vi "HFRR ADV v044.vi"() -> ()   [LabVIEW 2025] (continued)
                  n3206 = call-dynamic "Set Report Tab Width.vi"("report in"=w4016, "error in (no error)"=w4014) -> ("report out"=w4015:refnum<class "NI_report.lvclass">, "error out"=w4013:errorcluster)  [unwired: 12 in]
                }
                n3207 = local read "TITTLE"() -> (w3961:string)
                n3208 = call-dynamic "Set Report Header Text.vi"("report in"=w3944, "center header text"=w3961, "error in (no error)"=w3943) -> ("report out"=w3982:refnum<class "NI_report.lvclass">, "error out"=w3981:errorcluster)  [unwired: 11 in]
                n3209 = for {
                  N: 1 -> [_]
                  tunnel: [w4020] -> w3968
                  tunnel: [w4019] -> w3967
                  tunnel: w3982 -> [w4018]
                  tunnel: w3981 -> [w4017]
                  n3210 = call-dynamic "New Report Line.vi"("report in"=w4018, "error in (no error)"=w4017) -> ("report out"=w4020:refnum<class "NI_report.lvclass">, "error out"=w4019:errorcluster)  [unwired: 12 in]
                }
                n3211 = for {
                  N: 2 -> [_]
                  tunnel: [w4012] -> w3974
                  tunnel: [w4011] -> w3973
                  tunnel: w3968 -> [w4010]
                  tunnel: w3967 -> [w4009]
                  n3212 = call-dynamic "New Report Line.vi"("report in"=w4010, "error in (no error)"=w4009) -> ("report out"=w4012:refnum<class "NI_report.lvclass">, "error out"=w4011:errorcluster)  [unwired: 12 in]
                }
                n3213 = for {
                  N: 25 -> [_]
                  tunnel: w3974 -> [w4008]
                  tunnel: w3973 -> [w4006]
                  tunnel: [w4007] -> w3977
                  tunnel: [w4005] -> w3976
                  n3214 = call-dynamic "Set Report Tab Width.vi"("report in"=w4008, "error in (no error)"=w4006) -> ("report out"=w4007:refnum<class "NI_report.lvclass">, "error out"=w4005:errorcluster)  [unwired: 12 in]
                }
                n3215 = control-ref of="Tab Control 9"() -> (w3972:refnum<vi>)
                n3216 = call-dynamic "Append Control Image to Report.vi"("report in"=w3977, "alignment (default)"=HTML_Report_Image_Alignment."ABSMIDDLE", "ctrl reference"=w3972, "error in (no error)"=w3976) -> ("report out"=w3971:refnum<class "NI_report.lvclass">, "error out"=w3970:errorcluster)  [unwired: 8 in, 2 out]
                n3217 = for {
                  N: 3 -> [_]
                  tunnel: [w4004] -> w3955
                  tunnel: [w4003] -> w3954
                  tunnel: w3971 -> [w4002]
                  tunnel: w3970 -> [w4001]
                  n3218 = call-dynamic "New Report Line.vi"("report in"=w4002, "error in (no error)"=w4001) -> ("report out"=w4004:refnum<class "NI_report.lvclass">, "error out"=w4003:errorcluster)  [unwired: 12 in]
                }
                n3219 = for {
                  N: 100 -> [_]
                  tunnel: w3955 -> [w4000]
                  tunnel: w3954 -> [w3998]
                  tunnel: [w3999] -> w3951
                  tunnel: [w3997] -> w3949
                  n3220 = call-dynamic "Set Report Tab Width.vi"("report in"=w4000, "error in (no error)"=w3998) -> ("report out"=w3999:refnum<class "NI_report.lvclass">, "error out"=w3997:errorcluster)  [unwired: 12 in]
                }
                n3221 = String To Path(string="C:\\LAB-IQ\\im\\Temp_resized.jpg") -> (path=w3941:path)
                n3222 = call-poly <vilib>:"Append Image to Report.vi"("report in"=w3951, "path or URL of image"=w3941, "error in (no error)"=w3949) -> ("report out"=w3950:refnum<class "NI_report.lvclass">, "error out"=w3948:errorcluster)  [unwired: 9 in, 2 out]
                n3223 = call-poly <vilib>:"Open HTML Report in Browser.vi"("report in"=w3950, "error in (no error)"=w3948) -> ("report out"=w3985:refnum<class "NI_report.lvclass">, "error out"=w3984:errorcluster)  [unwired: 11 in, 1 out]
                n3224 = call-dynamic "Dispose Report.vi"("report in"=w3985, "error in (no error)"=w3984) -> ()  [unwired: 13 in, 1 out]
              }
              frame #2 {
              }
              frame #3 {
                n3225 = disable-structure shown="Disabled" {
                  frame Disabled {
                    n3226 = local read "String 10"() -> (w4025:string)
                    n3227 = Concatenate Strings("C:\\LAB-IQ-NXT\\Data\\" ("string"), w4025, ".jpg" ("string")) -> (w4023:string)
                    n3228 = String To Path(string=w4023) -> (path=w4022:path)
                    n3229 = Delete(path (use dialog)=w4022) -> ()  [unwired: 4 in, 3 out]
                  }
                  frame Enabled {
                  }
                }
                n3230 = local write "Print 2"(FALSE ("Print")) -> ()
              }
            }
          }
        }
      }
    }
    n3231 = Wait (ms)(milliseconds to wait=u32 50) -> ()  [unwired: 1 out]
    n3232 = Wait (ms)(milliseconds to wait=u32 50) -> ()  [unwired: 1 out]
    n3233 = local read "Quit"() -> (w2367:bool)
  }
  n3234 = VISA Close(VISA resource name=w46, error in (no error)=w45) -> ()  [unwired: 1 out]
  n3235 = while {
    stop <- w4176 stop-if-true
    n3236 = local read "Auto Start Test"() -> (w4174:bool)
    n3237 = local read "RUN"() -> (w4173:bool)
    n3238 = Wait (ms)(milliseconds to wait=u32 1000) -> ()  [unwired: 1 out]
    n3239 = Or(x=w4173, y=w4174) -> (x .or. y?=w4172:bool)
    n3240 = case shown="True" w4172 {
      frame False {
      }
      frame True {
        n3241 = local read "LVDT STROKE Actual"() -> (w4177:dbl)
        n3242 = In Range and Coerce(upper limit=1.2, x=w4177, lower limit=0.6) -> (In Range?=w4180:bool)  [unwired: 1 out]
        n3243 = call-poly <vilib>:"Random Number (Range).vi"("lower bound (0)"=0.998 ("upper bound (100)"), "upper bound (100)"=1.003) -> ("number"=w4178:dbl)  [unwired: 9 in]
        n3244 = case shown="True" w4180 {
          tunnel: [w4185 w4186] -> w4179
          tunnel: w4178 -> [_ w4186]
          tunnel: w4177 -> [w4185 _]
          frame False {
          }
          frame True {
          }
        }
        "LVDT STROKE DISPLAY" <- w4179
      }
    }
    n3245 = local read "Quit"() -> (w4176:bool)
  }
  n3246 = while {
    tunnel: [w4203] -> w54
    shift-right: [w4196] -> _
    shift-left: 0.0 -> [w4199]
    shift-right: [w4195] -> _
    shift-left: 0.0 -> [w4198]
    shift-right: [w4194] -> _
    shift-left: 100.0 ("vc_cmd") -> [w4197]
    stop <- w4203 stop-if-true
    # "PID LOGIC"
    n3247 = local read "run test Calibration"() -> (w4191:bool)
    n3248 = local read "RUN"() -> (w4201:bool)
    n3249 = local read "Auto Start Temp"() -> (w4192:bool)
    n3250 = local read "Auto Start Test"() -> (w4200:bool)
    n3251 = local read "START TEMP"() -> (w4190:bool)
    n3252 = And(x=w4192, y=w4200) -> (x .and. y?=w4193:bool)
    n3253 = Or(x=w4201, y=w4193) -> (x .or. y?=w4202:bool)
    n3254 = And(x=w4202, y=w4190) -> (x .and. y?=w4189:bool)
    n3255 = And(x=w4191, y=w4190) -> (x .and. y?=w4188:bool)
    n3256 = Or(x=w4188, y=w4189) -> (x .or. y?=w4187:bool)
    n3257 = Wait (ms)(milliseconds to wait="milliseconds to wait") -> ()  [unwired: 1 out]
    n3258 = case shown="True" w4187 {
      tunnel: [400.0 ("out_vc_cmd") w4222] -> w4194
      tunnel: [w4206 w4224] -> w4195
      tunnel: [w4206 w4223] -> w4196
      tunnel: w4199 -> [_ w4213]
      tunnel: w4198 -> [_ w4212]
      tunnel: w4197 -> [_ w4211]
      tunnel: w4191 -> [_ w4207]
      frame False {
        w4206 = 0.0 ("error_out")
      }
      frame True {
        n3259 = case shown="True" w4207 {
          tunnel: [w4231 1.0] -> w4209
          frame False {
            n3260 = local read "Set Strk"() -> (w4230:dbl)
            n3261 = Add(x=w4230, y="Add up Stroke") -> (x+y=w4231:dbl)
          }
          frame True {
          }
        }
        n3262 = local read "LVDT STROKE"() -> (w4208:dbl)
        n3263 = formula code="// Zero-Hardcode Explicit Positional-Form PID Engine\n// Inputs: target_stroke, measured_stroke, dt, prev_error, integral_accumulator_in, prev_vc_cmd\n//         kp, ki, kd, max_step_change, max_amplitude, min_amplitude, startup_cmd\n// Outputs: vc_cmd, error_out, out_error, integral_accumulator_out, out_vc_cmd\n\n// 1. Calculate Tracking Error\nfloat current_error = target_stroke - measured_stroke;\nerror_out = current_error;\n\n// 2. Compute Proportional Term\nfloat p_term = kp * current_error;\n\n// 3. Compute Derivative Term\nfloat d_term = 0.0;\nif (dt > 0.0) {\n    d_term = kd * ((current_error - prev_error) / dt);\n}\n\n// 4. Update and Accumulate Integral Term\nfloat current_integral = integral_accumulator_in + (current_error * dt);\nfloat i_term = ki * current_integral;\n\n// 5. Calculate Ideal Target Command (Anchored by startup baseline)\nfloat ideal_command = startup_cmd + p_term + i_term + d_term;\n\n// 6. Apply Loop Rate Limiting FIRST \n// (Forces the command to climb gradually from prev_vc_cmd instead of jumping straight to max)\nfloat raw_adjustment = ideal_command - prev_vc_cmd;\n\nif (raw_adjustment > max_step_change) {\n    raw_adjustment = max_step_change;\n} else if (raw_adjustment < -max_step_change) {\n    raw_adjustment = -max_step_change;\n}\n\nfloat next_vc_cmd = prev_vc_cmd + raw_adjustment;\n\n// 7. Anti-Windup Protection & Final Output Safety Safeguard Clamping\n// (Back-calculating based on what we are ACTUALLY outputting)\nif (next_vc_cmd > max_amplitude) {\n    float excess = next_vc_cmd - max_amplitude;\n    if (ki > 0.0) {\n        current_integral -= excess / ki;\n    }\n    next_vc_cmd = max_amplitude;\n} else if (next_vc_cmd < min_amplitude) {\n    float excess = next_vc_cmd - min_amplitude;\n    if (ki > 0.0) {\n        current_integral -= excess / ki;\n    }\n    next_vc_cmd = min_amplitude;\n}\n\n// 8. Map to Shift Registers for memory persistence\nvc_cmd = next_vc_cmd;\nout_error = current_error;                   \nintegral_accumulator_out = current_integral;  \nout_vc_cmd = next_vc_cmd;"("target_stroke"=w4209, "measured_stroke"=w4208, "dt"="dt", "integral_accumulator_in"=w4212, "prev_error"=w4213, "prev_vc_cmd"=w4211, "kp"="kp", "ki"="ki", "kd"="kd", "max_step_change"="max_step_change", "max_amplitude"="max_amplitude", "min_amplitude"="min_amplitude", "startup_cmd"="startup_cmd") -> ("vc_cmd"=w4228:dbl, "out_error"=w4223:dbl, "integral_accumulator_out"=w4224:dbl, "out_vc_cmd"=w4222:dbl)  [unwired: 1 out]
        "output Vpp" <- w4228
        n3264 = Number To Fractional String(number=w4228, precision (6)=i16 1) -> (F-format string=w4226:string)  [unwired: 2 in]
        n3265 = Concatenate Strings("DAC;" ("string"), w4226) -> (w4210:string)
        n3266 = local write "Due Write"(w4210) -> ()
        "prev_error" <- w4213
        "integral_accumulator_in" <- w4212
        "prev_vc_cmd" <- w4211
      }
    }
    n3267 = local read "Quit"() -> (w4203:bool)
  }
  n3268 = Or(x=w50, y=w49) -> (x .or. y?=w51:bool)
  n3269 = Or(x=w47, y=w51) -> (x .or. y?=w56:bool)
  n3270 = control-ref of="new picture"() -> ()  [unwired: 1 out]
  n3271 = Or(x=w59, y=w56) -> (x .or. y?=w53:bool)
  n3272 = Or(x=w53, y=w54) -> (x .or. y?=w48:bool)
  n3273 = while {
    tunnel: [w4233] -> w58
    i -> [w4240]
    stop <- w4233 stop-if-true
    n3274 = local read "Quit"() -> (w4233:bool)
    n3275 = Equal To 0?(x=w4240) -> (x = 0?=w4238:bool)
    n3276 = call "Elapsed Time3"("Time Target (s)"=45.0, "Auto Reset"=TRUE) -> ("Time has Elapsed"=w4237:bool)  [unwired: 10 in, 7 out]
    n3277 = Wait (ms)(milliseconds to wait=u32 50) -> ()  [unwired: 1 out]
    n3278 = Or(x=w4237, y=w4238) -> (x .or. y?=w4239:bool)
    n3279 = case shown="True" w4239 {
      frame False {
      }
      frame True {
        n3280 = call <vilib>:"System Exec.vi"("run minimized? (F)"=TRUE, "error in (no error)"="error in (no error)", "command line"="powercfg.exe -change -monitor-timeout-ac 0") -> ("error out"=w4251:errorcluster)  [unwired: 5 in, 3 out]
        n3281 = call <vilib>:"System Exec.vi"("run minimized? (F)"=TRUE, "error in (no error)"=w4251, "command line"="powercfg.exe -change -disk-timeout-ac 0") -> ("error out"=w4250:errorcluster)  [unwired: 5 in, 3 out]
        n3282 = call <vilib>:"System Exec.vi"("run minimized? (F)"=TRUE, "error in (no error)"=w4250, "command line"="powercfg.exe -change -standby-timeout-ac 0") -> ("error out"=w4249:errorcluster)  [unwired: 5 in, 3 out]
        n3283 = call <vilib>:"System Exec.vi"("run minimized? (F)"=TRUE, "error in (no error)"=w4249, "command line"="powercfg.exe -change -hibernate-timeout-ac 0") -> ("error out"=w4248:errorcluster)  [unwired: 5 in, 3 out]
        n3284 = call <vilib>:"Simple Error Handler.vi"("error in (no error)"=w4248) -> ("error out"=w4254:errorcluster)  [unwired: 4 in, 4 out]
        n3285 = call <vilib>:"Clear Errors.vi"("error in (no error)"=w4254) -> ("error out"=→"error out":errorcluster)  [unwired: 5 in, 1 out]
      }
    }
  }
  n3286 = Compound Arithmetic op=OR(w61, w48, w58) -> (w60:bool)
  n3287 = flat-sequence {
    tunnel: w60 -> [_]
    tunnel: [w4256] -> w30
    tunnel: w30 -> [_]
    frame #0 {
      n3288 = call "CLOSE CONNECTION.vi"() -> ("error out"=w4256:errorcluster)  [unwired: 11 in]
    }
    frame #1 {
      n3289 = Quit LabVIEW(quit? (T)=TRUE) -> ()
      n3290 = local write "Quit"(FALSE ("EXIT")) -> ()
    }
  }
  n3291 = property on="Heater Button" class="Bool (strict)"("Visible"=TRUE) -> ()  [unwired: 2 in, 2 out]
  n3292 = while {
    tunnel: [w4263] -> _
    i -> [w4263]
    stop <- w4259 stop-if-true
    # "Langauage selection"
    n3293 = Equal?(x="Lan flag", y=22.0) -> ()  [unwired: 1 out]
    n3294 = disable-structure shown="Disabled" {
      frame Disabled {
        n3295 = stacked-sequence {
          frame #0 {
            n3296 = case shown="\"Russian\"" "Language Selection" {
              tunnel: [0 1] -> w4265
              frame "English", Default {
              }
              frame "Russian" {
              }
            }
            n3297 = for {
              N: 130 -> [_]
              tunnel: "Table" -> [w4274]
              tunnel: w4265 -> [w4273]
              i -> [w4272]
              n3298 = Index Array(array=w4274, index (row)=w4272, index (col)=w4273) -> (element=w4271:string)
              n3299 = case shown="1" w4272 {
                tunnel: w4271 -> [w4275 w4276 _ w4277 w4278 w4279 w4280 w4281 w4282 w4283 w4284 w4285 w4286 w4287 w4288 w4289 w4290 w4291 w4292 w4293 w4294 w4295 w4296 w4297 w4298 w4299 w4300 w4301 w4302 _ _ w4303 w4304 w4305 w4306 w4307 w4308 w4317 w4324 w4331 w4338 w4342 w4345 w4348 w4350 w4352 w4353 w4354 w4355 w4356 w4357 w4358 w4359 w4360 w4361 w4362 w4363 w4364 w4365 w4366 w4367 w4368 w4369 w4370 w4371 w4372 w4373 w4374 w4375 w4376 w4377 w4378 w4379 w4380 w4381 w4382 w4383 w4384 w4385 w4386 w4387 w4388 w4389 w4390 w4391 w4392 w4393 w4394 w4395 w4396 w4397 w4398 w4399 w4400 w4401 w4402 w4403 w4404 w4405 w4406 w4407 w4408 w4409 w4410 w4411 _ w4412 w4413 w4414 w4415 w4416 w4417 w4418 w4419 w4420 w4421 w4422 w4423 w4424 _ w4425 w4426 w4427 w4428 w4429 w4430 _]
                frame 0 {
                  n3300 = local write "S"(w4275) -> ()
                }
                frame 1 {
                  n3301 = local write "S 2"(w4276) -> ()
                }
                frame 2 {
                }
                frame 3 {
                  n3302 = local write "S 4"(w4277) -> ()
                }
                frame 4 {
                  n3303 = property on="FILE" class="Str"("Caption.Text"=w4278) -> ()  [unwired: 2 in, 2 out]
                }
                frame 5 {
                  n3304 = property on="Fuel Discription :" class="Str"("Caption.Text"=w4279) -> ()  [unwired: 2 in, 2 out]
                }
                frame 6 {
                  n3305 = property on="Remarks :" class="Str"("Caption.Text"=w4280) -> ()  [unwired: 2 in, 2 out]
                }
                frame 7 {
                  n3306 = property on="Save & Continue" class="Bool (strict)"("Boolean Text.Text"=w4281) -> ()  [unwired: 2 in, 2 out]
                }
                frame 8 {
                }
                frame 9 {
                  n3307 = property on="Set Hz" class="DigNum (strict)"("Caption.Text"=w4283) -> ()  [unwired: 2 in, 2 out]
                }
                frame 10 {
                }
                frame 11 {
                  n3308 = property on="NORMAL LOAD" class="DigNum (strict)"("Caption.Text"=w4285) -> ()  [unwired: 2 in, 2 out]
                }
                frame 12 {
                }
                frame 13 {
                  n3309 = property on="Set Temp" class="DigNum (strict)"("Caption.Text"=w4287) -> ()  [unwired: 2 in, 2 out]
                }
                frame 14 {
                  n3310 = local write "S 15"(w4288) -> ()
                }
                frame 15 {
                  n3311 = property on="Set Rh" class="DigNum (strict)"("Caption.Text"=w4289) -> ()  [unwired: 2 in, 2 out]
                }
                frame 16 {
                }
                frame 17 {
                  n3312 = local write "S 18"(w4291) -> ()
                }
                frame 18 {
                  "String 17" <- w4292
                }
                frame 19 {
                  n3313 = property on="test time" class="DigNum (strict)"("Caption.Text"=w4293) -> ()  [unwired: 2 in, 2 out]
                }
                frame 20 {
                  "String 18" <- w4294
                  "String 22" <- w4294
                }
                frame 21 {
                  n3314 = property on="Elapsed time" class="DigNum (strict)"("Caption.Text"=w4295) -> ()  [unwired: 2 in, 2 out]
                }
                frame 22 {
                  n3315 = property on="Samplingtime 2" class="DigNum (strict)"("Caption.Text"=w4296) -> ()  [unwired: 2 in, 2 out]
                }
                frame 23 {
                  "String 21" <- w4297
                }
                frame 24 {
                  n3316 = property on="Countdown" class="DigNum (strict)"("Caption.Text"=w4298) -> ()  [unwired: 2 in, 2 out]
                }
                frame 25 {
                  n3317 = property on="Countdown 2" class="DigNum (strict)"("Caption.Text"=w4299) -> ()  [unwired: 2 in, 2 out]
                }
                frame 26 {
                  n3318 = property on="Engage" class="Bool (strict)"("Boolean Text.Text"=w4300) -> ()  [unwired: 2 in, 2 out]
                }
                frame 27 {
                  n3319 = property on="Boolean  4" class="Bool (strict)"("Boolean Text.Text"=w4301) -> ()  [unwired: 2 in, 2 out]
                }
                frame 28 {
                  n3320 = property on="Test \nStatus" class="Bool (strict)"("Boolean Text.Text"=w4302) -> ()  [unwired: 2 in, 2 out]
                }
                frame 29 {
                }
                frame 30 {
                }
                frame 31 {
                }
                frame 32 {
                  n3321 = property on="RSTCOF" class="Bool"("Boolean Text.Text"=w4304) -> ()  [unwired: 2 in, 2 out]
                  n3322 = property on="RST FF" class="Bool"("Boolean Text.Text"=w4304) -> ()  [unwired: 2 in, 2 out]
                  n3323 = property on="RST TEMP" class="Bool"("Boolean Text.Text"=w4304) -> ()  [unwired: 2 in, 2 out]
                  n3324 = property on="RSTV1 3" class="Bool"("Boolean Text.Text"=w4304) -> ()  [unwired: 2 in, 2 out]
                  n3325 = property on="rstv2" class="Bool"("Boolean Text.Text"=w4304) -> ()  [unwired: 2 in, 2 out]
                  n3326 = property on="RSTV1 2" class="Bool"("Boolean Text.Text"=w4304) -> ()  [unwired: 2 in, 2 out]
                  n3327 = property on="RST CP" class="Bool"("Boolean Text.Text"=w4304) -> ()  [unwired: 2 in, 2 out]
                }
                frame 33 {
                  "S 61" <- w4305
                }
                frame 34 {
                  "String 23" <- w4306
                }
                frame 35 {
                  n3328 = property on="Rh Before" class="DigNum (strict)"("Caption.Text"=w4307) -> ()  [unwired: 2 in, 2 out]
                }
                frame 36 {
                  n3329 = Match Pattern(string=w4308, regular expression=",") -> (before substring=→"bs":string, after substring=→"as":string)  [unwired: 1 in, 2 out]
                  n3330 = property on="Rh After" class="DigNum (strict)"("Caption.Text"=w4308) -> ()  [unwired: 2 in, 2 out]
                }
                frame 37 {
                  n3331 = Match Pattern(string=w4317, regular expression=",") -> (before substring=w4316:string, after substring=w4315:string)  [unwired: 1 in, 2 out]
                  "bs" <- w4316
                  "as" <- w4315
                  n3332 = Concatenate Strings(w4316, w4315) -> (w4312:string)
                  n3333 = property on="Humidity before test 2" class="DigNum (strict)"("Caption.Text"=w4312) -> ()  [unwired: 2 in, 2 out]
                  n3334 = Concatenate Strings(w4312, "=" ("string")) -> (w4313:string)
                  n3335 = local write "S 38"(w4313) -> ()
                }
                frame 38 {
                  n3336 = Match Pattern(string=w4324, regular expression=",") -> (before substring=w4323:string, after substring=w4322:string)  [unwired: 1 in, 2 out]
                  "bs" <- w4323
                  "as" <- w4322
                  n3337 = Concatenate Strings(w4323, w4322) -> (w4319:string)
                  n3338 = property on="Humidity after test 2" class="DigNum (strict)"("Caption.Text"=w4319) -> ()  [unwired: 2 in, 2 out]
                  n3339 = Concatenate Strings(w4319, "=" ("string")) -> (w4321:string)
                  n3340 = local write "S 39"(w4321) -> ()
                }
                frame 39 {
                  n3341 = Match Pattern(string=w4331, regular expression=",") -> (before substring=w4330:string, after substring=w4329:string)  [unwired: 1 in, 2 out]
                  "bs" <- w4330
                  "as" <- w4329
                  n3342 = Concatenate Strings(w4330, w4329) -> (w4326:string)
                  n3343 = property on="Temperature before test 2" class="DigNum (strict)"("Caption.Text"=w4326) -> ()  [unwired: 2 in, 2 out]
                  n3344 = Concatenate Strings(w4326, "=" ("string")) -> (→"String 34":string)
                }
                frame 40 {
                  n3345 = Match Pattern(string=w4338, regular expression=",") -> (before substring=w4337:string, after substring=w4336:string)  [unwired: 1 in, 2 out]
                  "bs" <- w4337
                  "as" <- w4336
                  n3346 = Concatenate Strings(w4337, w4336) -> (w4333:string)
                  n3347 = property on="Temperature after test 2" class="DigNum (strict)"("Caption.Text"=w4333) -> ()  [unwired: 2 in, 2 out]
                  n3348 = Concatenate Strings(w4333, "=" ("string")) -> (→"String 35":string)
                  n3349 = property on="Temperature after test" class="DigNum (strict)"("Caption.Text"=w4333) -> ()  [unwired: 2 in, 2 out]
                }
                frame 41 {
                  n3350 = property on="AVP 2" class="DigNum (strict)"("Caption.Text"=w4342) -> ()  [unwired: 2 in, 2 out]
                  n3351 = Concatenate Strings(w4342, "=" ("string")) -> (→"String 36":string)
                }
                frame 42 {
                  n3352 = property on="MWSD 2" class="DigNum (strict)"("Caption.Text"=w4345) -> ()  [unwired: 2 in, 2 out]
                  n3353 = Concatenate Strings(w4345, "=" ("string")) -> (→"String 37":string)
                }
                frame 43 {
                  n3354 = property on="HCF 2" class="DigNum (strict)"("Caption.Text"=w4348) -> ()  [unwired: 2 in, 2 out]
                  n3355 = Concatenate Strings(w4348, "=" ("string")) -> (→"String 38":string)
                }
                frame 44 {
                  n3356 = Concatenate Strings(w4350, "=" ("string")) -> (→"String 39":string)
                  n3357 = property on="WS1.4 2" class="DigNum (strict)"("Caption.Text"=w4350) -> ()  [unwired: 2 in, 2 out]
                }
                frame 45 {
                }
                frame 46 {
                  n3358 = local write "S 47"(w4353) -> ()
                }
                frame 47 {
                  n3359 = local write "S 48"(w4354) -> ()
                }
                frame 48 {
                  n3360 = local write "S 49"(w4355) -> ()
                }
                frame 49 {
                  n3361 = local write "S 50"(w4356) -> ()
                }
                frame 50 {
                  n3362 = local write "S 51"(w4357) -> ()
                }
                frame 51 {
                  n3363 = local write "S 52"(w4358) -> ()
                }
                frame 52 {
                  n3364 = local write "S 53"(w4359) -> ()
                }
                frame 53 {
                  n3365 = local write "S 54"(w4360) -> ()
                }
                frame 54 {
                  n3366 = local write "S 55"(w4361) -> ()
                }
                frame 55 {
                  n3367 = local write "S 56"(w4362) -> ()
                }
                frame 56 {
                  n3368 = local write "S 57"(w4363) -> ()
                }
                frame 57 {
                  n3369 = local write "S 58"(w4364) -> ()
                }
                frame 58 {
                  n3370 = local write "S 59"(w4365) -> ()
                }
                frame 59 {
                  n3371 = local write "S 60"(w4366) -> ()
                }
                frame 60 {
                  n3372 = local write "S 62"(w4367) -> ()
                }
                frame 61 {
                  n3373 = local write "S 63"(w4368) -> ()
                }
                frame 62 {
                  n3374 = local write "S 64"(w4369) -> ()
                }
                frame 63 {
                  n3375 = local write "S 65"(w4370) -> ()
                }
                frame 64 {
                  n3376 = local write "S 66"(w4371) -> ()
                }
                frame 65 {
                  n3377 = local write "S 67"(w4372) -> ()
                }
                frame 66 {
                  n3378 = local write "S 68"(w4373) -> ()
                }
                frame 67 {
                  n3379 = local write "S 69"(w4374) -> ()
                }
                frame 68 {
                  n3380 = local write "S 70"(w4375) -> ()
                }
                frame 69 {
                  n3381 = local write "S 71"(w4376) -> ()
                }
                frame 70 {
                  n3382 = local write "S 72"(w4377) -> ()
                }
                frame 71 {
                  n3383 = local write "S 73"(w4378) -> ()
                }
                frame 72 {
                  n3384 = local write "S 74"(w4379) -> ()
                }
                frame 73 {
                  n3385 = local write "S 75"(w4380) -> ()
                }
                frame 74 {
                  n3386 = local write "S 76"(w4381) -> ()
                }
                frame 75 {
                  n3387 = local write "S 77"(w4382) -> ()
                }
                frame 76 {
                  n3388 = local write "S 78"(w4383) -> ()
                }
                frame 77 {
                  n3389 = local write "S 79"(w4384) -> ()
                }
                frame 79 {
                  n3390 = property on="Sample Temperature ( °C )" class="XYGraph (strict)"("Y Scale.Name Label.Text"=w4385) -> ()  [unwired: 2 in, 2 out]
                }
                frame 80 {
                  n3391 = local write "S 81"(w4386) -> ()
                  n3392 = property on="Humidity ( %RH )" class="XYGraph (strict)"("Y Scale.Name Label.Text"=w4386) -> ()  [unwired: 2 in, 2 out]
                }
                frame 78 {
                  n3393 = property on="Air Temperature  ( °C )" class="XYGraph (strict)"("X Scale.Name Label.Text"=w4387) -> ()  [unwired: 2 in, 2 out]
                  n3394 = property on="Humidity ( %RH )" class="XYGraph (strict)"("X Scale.Name Label.Text"=w4387) -> ()  [unwired: 2 in, 2 out]
                  n3395 = property on="Sample Temperature ( °C )" class="XYGraph (strict)"("X Scale.Name Label.Text"=w4387) -> ()  [unwired: 2 in, 2 out]
                  n3396 = property on="Coefficient Of Friction" class="XYGraph (strict)"("X Scale.Name Label.Text"=w4387) -> ()  [unwired: 2 in, 2 out]
                }
                frame 81 {
                  n3397 = property on="Air Temperature  ( °C )" class="XYGraph (strict)"("Y Scale.Name Label.Text"=w4388) -> ()  [unwired: 2 in, 2 out]
                }
                frame 82 {
                  n3398 = local write "S 84"(w4389) -> ()
                }
                frame 83 {
                  n3399 = local write "S 85"(w4390) -> ()
                }
                frame 84 {
                  n3400 = local write "S 86"(w4391) -> ()
                }
                frame 85 {
                  n3401 = local write "S 87"(w4392) -> ()
                }
                frame 86 {
                  n3402 = local write "S 88"(w4393) -> ()
                }
                frame 87 {
                }
                frame 88 {
                  n3403 = local write "S 90"(w4395) -> ()
                }
                frame 89 {
                  n3404 = local write "S 91"(w4396) -> ()
                }
                frame 90 {
                  n3405 = local write "S 92"(w4397) -> ()
                }
                frame 91 {
                  n3406 = local write "S 93"(w4398) -> ()
                }
                frame 92 {
                  n3407 = local write "S 94"(w4399) -> ()
                }
                frame 93 {
                  n3408 = local write "S 95"(w4400) -> ()
                }
                frame 94 {
                  n3409 = local write "S 96"(w4401) -> ()
                }
                frame 95 {
                  n3410 = local write "S 97"(w4402) -> ()
                }
                frame 96 {
                  n3411 = local write "S 98"(w4403) -> ()
                }
                frame 97 {
                  n3412 = local write "S 99"(w4404) -> ()
                }
                frame 98 {
                  n3413 = local write "S 100"(w4405) -> ()
                }
                frame 99 {
                  n3414 = local write "S 101"(w4406) -> ()
                }
                frame 100 {
                  n3415 = local write "S 102"(w4407) -> ()
                }
                frame 101 {
                  n3416 = local write "S 103"(w4408) -> ()
                }
                frame 102 {
                  n3417 = local write "S 104"(w4409) -> ()
                }
                frame 103 {
                  n3418 = local write "S 105"(w4410) -> ()
                }
                frame 104 {
                  n3419 = local write "S 106"(w4411) -> ()
                }
                frame 105 {
                }
                frame 106 {
                  n3420 = property on="OK Button 17" class="Bool (strict)"("Boolean Text.Text"=w4412) -> ()  [unwired: 2 in, 2 out]
                }
                frame 107 {
                  n3421 = property on="OK Button 16" class="Bool (strict)"("Boolean Text.Text"=w4413) -> ()  [unwired: 2 in, 2 out]
                }
                frame 108 {
                  n3422 = property on="TITTLE" class="Str"("Caption.Text"=w4414) -> ()  [unwired: 2 in, 2 out]
                }
                frame 109 {
                  "String 30" <- w4415
                }
                frame 110 {
                  n3423 = property on="Test Date" class="Str"("Caption.Text"=w4416) -> ()  [unwired: 2 in, 2 out]
                  "String 31" <- w4416
                }
                frame 111 {
                  n3424 = property on="Sample ID" class="Str"("Caption.Text"=w4417) -> ()  [unwired: 2 in, 2 out]
                  "String 32" <- w4417
                }
                frame 112 {
                  n3425 = property on="Tested by" class="Str"("Caption.Text"=w4418) -> ()  [unwired: 2 in, 2 out]
                  "String 33" <- w4418
                }
                frame 113 {
                  n3426 = property on="System Configured Printers 2" class="Arr (strict)"("Caption.Text"=w4419) -> ()  [unwired: 2 in, 2 out]
                }
                frame 114 {
                  n3427 = property on="Selected Printer" class="Str"("Caption.Text"=w4420) -> ()  [unwired: 2 in, 2 out]
                }
                frame 115 {
                  n3428 = property on="Select Printer 3" class="DigNum (strict)"("Caption.Text"=w4421) -> ()  [unwired: 2 in, 2 out]
                }
                frame 116 {
                  n3429 = property on="Print" class="Bool (strict)"("Boolean Text.Text"=w4422) -> ()  [unwired: 2 in, 2 out]
                }
                frame 117 {
                  "String 41" <- w4423
                }
                frame 118 {
                  n3430 = property on="tested by" class="Str"("Caption.Text"=w4424) -> ()  [unwired: 2 in, 2 out]
                }
                frame 119 {
                }
                frame 120 {
                  n3431 = property on="Export" class="Bool (strict)"("Boolean Text.Text"=w4425) -> ()  [unwired: 2 in, 2 out]
                }
                frame 121 {
                }
                frame 122 {
                }
                frame 123 {
                  n3432 = property on="Select File Type" class="Enum (strict)"("Caption.Text"=w4428) -> ()  [unwired: 2 in, 2 out]
                }
                frame 124 {
                  n3433 = property on="s.NO" class="Str"("Caption.Text"=w4429) -> ()  [unwired: 2 in, 2 out]
                  "String 45" <- w4429
                }
                frame 125 {
                  n3434 = property on="trip1 8" class="Bool (strict)"("Boolean Text.Text"=w4430) -> ()  [unwired: 2 in, 2 out]
                }
                frame 126, Default {
                }
              }
            }
          }
          frame #1 {
            w4438 = TRUE ("Visible")
            n3435 = local read "S 91"() -> (w4455:string)
            n3436 = local read "S 90"() -> (w4454:string)
            n3437 = local read "S 88"() -> (w4453:string)
            n3438 = property on="File Path" class="Path"("Caption.Text"=w4454) -> ()  [unwired: 2 in, 2 out]
            n3439 = local read "S 71"() -> (w4448:string)
            n3440 = local read "S 86"() -> (w4450:string)
            n3441 = local read "S 85"() -> (w4451:string)
            n3442 = local read "S 87"() -> (w4449:string)
            n3443 = local read "S 84"() -> (w4452:string)
            n3444 = local read "S 103"() -> (w4437:string)
            n3445 = local read "S 104"() -> (w4436:string)
            n3446 = property on="Password" class="Str"("Caption.Text"=w4451) -> ()  [unwired: 2 in, 2 out]
            n3447 = property on="EDIT" class="Bool (strict)"("Boolean Text.Text"=w4448) -> ()  [unwired: 2 in, 2 out]
            n3448 = property on="SAVE" class="Bool (strict)"("Boolean Text.Text"=w4452) -> ()  [unwired: 2 in, 2 out]
            n3449 = Build Array(w4437, w4436) -> (w4435:string[])
            n3450 = property on="Heater Button" class="Bool (strict)"("Strings [4]"=w4435) -> ()  [unwired: 2 in, 2 out]
            n3451 = local read "S 92"() -> (w4447:string)
            n3452 = local read "S 93"() -> (w4446:string)
            n3453 = local read "S 105"() -> (w4433:string)
            n3454 = local read "S 106"() -> (w4432:string)
            n3455 = Build Array(w4447, w4446) -> ()  [unwired: 1 out]
            n3456 = Build Array(w4433, w4432) -> (w4434:string[])
            n3457 = local read "S 95"() -> (w4444:string)
            n3458 = local read "S 94"() -> (w4445:string)
            n3459 = local read "bs"() -> (w4460:string)
            n3460 = local read "as"() -> (w4461:string)
            n3461 = property on="Humidity" class="Bool (strict)"("Strings [4]"=w4434) -> ()  [unwired: 2 in, 2 out]
            n3462 = Concatenate Strings(w4460, "\r", w4461) -> ()  [unwired: 1 out]
            n3463 = property on="Rh After" class="DigNum (strict)"("Caption.Size to Text?"=TRUE ("Caption.Size to Text")) -> ()  [unwired: 2 in, 2 out]
            n3464 = local read "S 48"() -> (w4484:string)
            n3465 = local read "S 50"() -> (w4482:string)
            n3466 = local read "S 51"() -> (w4481:string)
            n3467 = local read "S 49"() -> (w4483:string)
            n3468 = local read "S 52"() -> (w4480:string)
            n3469 = local read "as"() -> (w4465:string)
            n3470 = local read "bs"() -> (w4466:string)
            n3471 = local read "S 56"() -> (w4479:string)
            n3472 = local read "S 57"() -> (w4478:string)
            n3473 = local read "S 58"() -> (w4477:string)
            n3474 = local read "S 59"() -> (w4476:string)
            n3475 = property on="OPEN" class="Bool (strict)"("Boolean Text.Text"=w4480) -> ()  [unwired: 2 in, 2 out]
            n3476 = property on="OPEN 1" class="Bool (strict)"("Boolean Text.Text"=w4484) -> ()  [unwired: 2 in, 2 out]
            n3477 = property on="OPEN 2" class="Bool (strict)"("Boolean Text.Text"=w4483) -> ()  [unwired: 2 in, 2 out]
            n3478 = property on="OPEN 3" class="Bool (strict)"("Boolean Text.Text"=w4482) -> ()  [unwired: 2 in, 2 out]
            n3479 = property on="OPEN 4" class="Bool (strict)"("Boolean Text.Text"=w4481) -> ()  [unwired: 2 in, 2 out]
            n3480 = Concatenate Strings(w4466, "\r", w4465) -> ()  [unwired: 1 out]
            n3481 = local read "S 102"() -> (w4439:string)
            n3482 = property on="КОФ1" class="DigNum (strict)"("Caption.Text"=w4479) -> ()  [unwired: 2 in, 2 out]
            n3483 = local read "S 98"() -> (w4443:string)
            n3484 = local read "S 99"() -> (w4442:string)
            n3485 = local read "S 100"() -> (w4441:string)
            n3486 = local read "S 101"() -> (w4440:string)
            n3487 = property on="КОФ2" class="DigNum (strict)"("Caption.Text"=w4478) -> ()  [unwired: 2 in, 2 out]
            n3488 = property on="КОФ3" class="DigNum (strict)"("Caption.Text"=w4477) -> ()  [unwired: 2 in, 2 out]
            n3489 = property on="КОФ4" class="DigNum (strict)"("Caption.Text"=w4476) -> ()  [unwired: 2 in, 2 out]
            n3490 = local read "bs"() -> (w4464:string)
            n3491 = local read "as"() -> (w4463:string)
            n3492 = local read "S 60"() -> (w4475:string)
            n3493 = local read "S 54"() -> (w4485:string)
            n3494 = Concatenate Strings(w4464, "\r", w4463) -> ()  [unwired: 1 out]
            n3495 = Concatenate Strings(w4485, w4475) -> ()  [unwired: 1 out]
            n3496 = local read "S 77"() -> (→"String 43":string)
            n3497 = local read "S 76"() -> (w4458:string)
            n3498 = local read "S 78"() -> (w4457:string)
            n3499 = local read "S 71"() -> (w4469:string)
            n3500 = local read "S 66"() -> (w4474:string)
            n3501 = local read "S 67"() -> (w4473:string)
            n3502 = local read "S 68"() -> (w4472:string)
            n3503 = local read "S 69"() -> (w4471:string)
            n3504 = local read "S 70"() -> (w4470:string)
            n3505 = property on="AIR TEMP" class="DigNum (strict)"("Caption.Text"=w4457) -> ()  [unwired: 2 in, 2 out]
            n3506 = property on="Set Strk" class="DigNum (strict)"("Caption.Text"=w4458) -> ()  [unwired: 2 in, 2 out]
            n3507 = property on="SPEED OUT:" class="DigNum (strict)"("Caption.Text"=w4472) -> ()  [unwired: 2 in, 2 out]
            n3508 = property on="EDIT" class="Bool (strict)"("Boolean Text.Text"=w4469) -> ()  [unwired: 2 in, 2 out]
            n3509 = local read "S 79"() -> (w4456:string)
          }
          frame #2 {
          }
        }
        n3510 = local write "Lan flag"(10.0 ("Lan flag")) -> ()
      }
      frame Enabled {
      }
    }
    n3511 = Wait (ms)(milliseconds to wait=u32 2000) -> ()  [unwired: 1 out]
    n3512 = local read "Quit"() -> (w4259:bool)
  }
  n3513 = while {
    shift-right: [w4491] -> _
    shift-left: _ -> [w4492]
    shift-right: [w4489] -> _
    shift-left: T18 {"Read Heave and Surge"="", "Bytes at Heave Port"=0.0, "Heave and Surge COM Port:"="COM9", "Com Port 2"="COM7", "Residual Due"="", "Heave COM Status 2"=TRUE, "Heave COM Status"=TRUE, "Port 2"=TRUE, "Sway PPR"=6400.0, "Surge PPR"=6400.0, "Heave PPR"=6400.0, "Sway Pitch"=2.0, "Surge Pitch"=3.0, "Heave Pitch"=4.0, "Sway Pulses/mm"=320.0, "Surge Pulses/mm"=1600.0, "Heave Pulses/mm"=1600.0, "inner loop"=0.0, "Read Heave and Surge 2"="", "String 36"="", "Write S"=FALSE, "WriteCC1"=[""], "Heave COM Loop"=0, "LastCom"="", "EXIT"=FALSE, "Error Heave"={"status"=TRUE, "code"=-1073807343, "source"=""}} -> [w4488]
    shift-right: [w4486] -> _
    shift-left: enum16{"init", "MAIN", "Panel Close"}."init" -> [w4487]
    stop <- w4490 stop-if-true
    # "HUMIDITY LOOP LOGIC"
    n3514 = case shown="\"MAIN\"" w4487 {
      tunnel: w4492 -> [w4506 w4530 w4594 w4596]
      tunnel: [w4501 w4517 w4594 w4596] -> w4491
      tunnel: [_ _ TRUE _] -> w4490
      tunnel: [w4498 w4515 w4592 w4595] -> w4489
      tunnel: w4488 -> [w4503 w4529 w4592 w4595]
      tunnel: [enum16{"init", "MAIN", "Panel Close"}."MAIN" w4524 _ _] -> w4486
      frame "init" {
        n3515 = local read "C3 :"() -> (w4493:refnum<visa-resource-name>)
        n3516 = Bundle By Name(cluster=w4503, "Heave and Surge COM Port:"=w4493) -> (w4502:T18)
        n3517 = call "Instrument fgv uno.vi"("Enum"=T31."INIT", "error in (no error) 2"=w4506, "INPUT"=w4502) -> ("error"=w4504:errorcluster, "output"=w4500:T18)  [unwired: 6 in, 1 out]
        n3518 = case shown="Error" w4504 {
          selector: w4504 -> [w4508 _]
          tunnel: [w4508 w4512] -> w4501
          tunnel: w4500 -> [w4507 w4510]
          tunnel: [w4507 w4509] -> w4499
          frame No Error {
          }
          frame Error {
            n3519 = call "Instrument fgv uno.vi"("Enum"=T31."ERROR INIT", "INPUT"=w4510) -> ("error"=w4513:errorcluster, "output"=w4509:T18)  [unwired: 7 in, 1 out]
            n3520 = call <vilib>:"Clear Errors.vi"("error in (no error)"=w4513) -> ("error out"=w4512:errorcluster)  [unwired: 5 in, 1 out]
          }
        }
        n3521 = local read "LastCom Humidity"() -> (w4496:string)
        n3522 = Unbundle By Name(w4499) -> ("Heave COM Status 2"=→"COM Status":bool, "Error Heave"=→"Error":errorcluster)  [unwired: 1 out]
        n3523 = Bundle By Name(cluster=w4499, "LastCom"=w4496) -> (w4498:T18)
      }
      frame "MAIN" {
        n3524 = Unbundle By Name(w4529) -> ("Com Port 2"=w4519:refnum<visa-resource-name>)
        n3525 = local read "C3 :"() -> (w4520:refnum<visa-resource-name>)
        n3526 = local write "COM Port Humidity :"(w4519) -> ()
        n3527 = Bundle By Name(cluster=w4529, "Heave and Surge COM Port:"=w4520) -> (w4528:T18)
        n3528 = Equal?(x=w4519, y=w4520) -> (x = y?=w4533:bool)
        n3529 = case shown="True" w4533 {
          tunnel: [w4548 w4565] -> w4518
          tunnel: w4530 -> [w4549 w4571]
          tunnel: w4528 -> [w4547 w4569]
          tunnel: [w4546 w4564] -> w4516
          frame False {
            n3530 = call <vilib>:"Clear Errors.vi"("error in (no error)"=w4549) -> ("error out"=w4545:errorcluster)  [unwired: 5 in, 1 out]
            n3531 = call "Instrument fgv uno.vi"("Enum"=T31."ERROR INIT", "error in (no error) 2"=w4545, "INPUT"=w4547) -> ("error"=w4551:errorcluster, "output"=w4546:T18)  [unwired: 6 in, 1 out]
            n3532 = call <vilib>:"Clear Errors.vi"("error in (no error)"=w4551) -> ("error out"=w4548:errorcluster)  [unwired: 5 in, 1 out]
          }
          frame True {
            n3533 = call "Instrument fgv uno.vi"("Enum"=T31."READ", "error in (no error) 2"=w4571, "INPUT"=w4569) -> ("error"=w4570:errorcluster, "output"=w4563:T18)  [unwired: 6 in, 1 out]
            n3534 = Bundle By Name(cluster=w4563, "String 36"="WRITE HUMIDITY") -> (w4562:T18)
            n3535 = case shown="True" "Write Humidity" {
              selector: "Write Humidity" -> [_ w4591]
              tunnel: w4570 -> [w4584 w4590]
              tunnel: [w4584 w4589] -> w4560
              tunnel: w4562 -> [w4583 w4587]
              tunnel: [w4583 w4586] -> w4559
              frame False {
              }
              frame True {
                n3536 = Not(x=w4591) -> (.not. x?=w4585:bool)
                n3537 = local write "Write Humidity"(w4585) -> ()
                n3538 = call "Instrument fgv uno.vi"("Enum"=T31."MANUAL WRITE", "error in (no error) 2"=w4590, "INPUT"=w4587) -> ("error"=w4589:errorcluster, "output"=w4586:T18)  [unwired: 6 in, 1 out]
              }
            }
            n3539 = Array Size(array="WriteHumidity") -> (size(s)=w4557:i32)
            n3540 = Greater Than 0?(x=w4557) -> (x > 0?=w4556:bool)
            n3541 = call "Instrument fgv uno.vi"("Enum"=T31."WRITE", "error in (no error) 2"=w4560, "WriteCC1"="WriteHumidity", "INPUT"=w4559) -> ("error"=w4567:errorcluster, "WriteCC1 2"=w4558:string[], "output"=w4566:T18)  [unwired: 5 in]
            n3542 = case shown="True" w4556 {
              tunnel: w4558 -> [_ w4573]
              frame False {
              }
              frame True {
                n3543 = local write "WriteHumidity"(w4573) -> ()
              }
            }
            n3544 = case shown="No Error" w4567 {
              selector: w4567 -> [w4574 w4577]
              tunnel: w4566 -> [w4575 w4582]
              tunnel: [w4575 w4581] -> w4564
              tunnel: [w4574 w4579] -> w4565
              frame No Error {
              }
              frame Error {
                n3545 = call <vilib>:"Clear Errors.vi"("error in (no error)"=w4577) -> ("error out"=w4576:errorcluster)  [unwired: 5 in, 1 out]
                n3546 = call "Instrument fgv uno.vi"("Enum"=T31."ERROR INIT", "error in (no error) 2"=w4576, "INPUT"=w4582) -> ("error"=w4580:errorcluster, "output"=w4581:T18)  [unwired: 6 in, 1 out]
                n3547 = call <vilib>:"Clear Errors.vi"("error in (no error)"=w4580) -> ("error out"=w4579:errorcluster)  [unwired: 5 in, 1 out]
              }
            }
            n3548 = Unbundle By Name(w4564) -> ("LastCom"=→"LastCom Humidity":string, "Read Heave and Surge"=→"Read HUMIDITY":string)
          }
        }
        n3549 = Unbundle By Name(w4516) -> ("Heave COM Status 2"=w4532:bool, "Error Heave"=w4521:errorcluster, "Bytes at Heave Port"=→"Bytes at Humidity Port  2":dbl)  [unwired: 1 out]
        n3550 = Unbundle By Name(w4521) -> ("status"=→"Humidity Port":bool)
        n3551 = Not(x=w4532) -> (.not. x?=w4522:bool)
        n3552 = local write "Error"(w4521) -> ()
        n3553 = local read "Quit"() -> (w4525:bool)
        n3554 = local write "COM Status"(w4522) -> ()
        n3555 = Select(t=enum16{"init", "MAIN", "Panel Close"}."Panel Close", s=w4525, f=enum16{"init", "MAIN", "Panel Close"}."MAIN") -> (s? t:f=w4524:enum16{"init", "MAIN", "Panel Close"})
        n3556 = local read "Humidity 2"() -> (w4514:bool)
        n3557 = case shown="True" w4514 {
          selector: w4514 -> [_ w4536]
          tunnel: w4518 -> [w4534 w4541]
          tunnel: [w4534 w4540] -> w4517
          tunnel: w4516 -> [w4535 w4539]
          tunnel: [w4535 w4538] -> w4515
          frame False {
          }
          frame True {
            n3558 = Not(x=w4536) -> (.not. x?=→"Humidity 2":bool)
            n3559 = call <vilib>:"Clear Errors.vi"("error in (no error)"=w4541) -> ("error out"=w4544:errorcluster)  [unwired: 5 in, 1 out]
            n3560 = call "Instrument fgv uno.vi"("Enum"=T31."ERROR INIT", "error in (no error) 2"=w4544, "INPUT"=w4539) -> ("error"=w4542:errorcluster, "output"=w4538:T18)  [unwired: 6 in, 1 out]
            n3561 = call <vilib>:"Clear Errors.vi"("error in (no error)"=w4542) -> ("error out"=w4540:errorcluster)  [unwired: 5 in, 1 out]
          }
        }
      }
      frame "Panel Close" {
      }
      frame Default {
      }
    }
  }
  n3562 = while {
    stop <- w4598 stop-if-true
    n3563 = call <vilib>:"High Resolution Polling Wait.vi"("seconds to wait"=0.05) -> ()  [unwired: 10 in, 1 out]
    n3564 = disable-structure shown="Enabled" {
      frame Disabled {
        n3565 = local read "Read HUMIDITY"() -> (w4599:string)
        n3566 = Spreadsheet String To Array(delimiter (Tab)=",", format string="", spreadsheet string=w4599, array type (2D Dbl)=string[] []) -> (array=w4618:string[])
        n3567 = for {
          tunnel: w4618 -> [w4627] mode=indexing
          tunnel: string[] ["STATE;", "SET;", "RH;", "T;", "AMB_RH;", "AMB_T;", "PUMP;", "FAN_IN;", "FAN_OUT;", "DEHUM;", "CURRENT;", "STALL;"] -> [w4626] mode=indexing
          tunnel: [w4625] -> w4617 mode=indexing
          n3568 = Match Pattern(string=w4627, regular expression=w4626) -> (after substring=w4625:string)  [unwired: 1 in, 3 out]
        }
        n3569 = Index Array(array=w4617) -> (element #1=w4616:string, element #2=w4615:string, element #3=w4607:string, element #4=w4606:string, element #5=w4605:string, element #6=w4614:string, element #7=w4613:string, element #8=w4612:string, element #9=w4611:string, element #10=w4610:string, element #11=w4609:string, element #12=w4608:string)  [unwired: 12 in]
        n3570 = Fract/Exp String To Number(string=w4607) -> (number=w4600:dbl)  [unwired: 3 in, 1 out]
        n3571 = Fract/Exp String To Number(string=w4605) -> (number=w4604:dbl)  [unwired: 3 in, 1 out]
        n3572 = local write "Ambient Humidity :"(w4604) -> ()
        n3573 = Equal?(x=w4600, y=0.0) -> (x = y?=w4602:bool)
        n3574 = case shown="True" w4602 {
          tunnel: [w4623 w4624] -> w4601
          tunnel: w4600 -> [w4623 _]
          frame False {
            (unwired) 0.0
            "Humidity temp" <- w4623
          }
          frame True {
            n3575 = local read "Humidity temp"() -> (w4624:dbl)
          }
        }
        "RH Numeric:" <- w4601
      }
      frame Enabled {
        n3576 = local read "Read HUMIDITY"() -> (w4647:string)
        n3577 = Spreadsheet String To Array(delimiter (Tab)=",", format string="", spreadsheet string=w4647, array type (2D Dbl)=dbl[] []) -> (array=w4643:dbl[])
        n3578 = Index Array(array=w4643) -> (element #1=→"STATE :":dbl, element #2=→"SET :":dbl, element #3=w4628:dbl, element #4=→"T :":dbl, element #5=→"AMB_RH :":dbl, element #6=→"AMB_T :":dbl, element #7=→"PUMP :":dbl, element #8=→"FAN_IN :":dbl, element #9=→"FAN_OUT :":dbl, element #10=→"DEHUM :":dbl, element #11=→"CURRENT :":dbl, element #12=→"STALL":dbl)  [unwired: 12 in]
        "RH :" <- w4628
        n3579 = Equal?(x=w4628, y=0.0) -> (x = y?=w4631:bool)
        n3580 = case shown="False" w4631 {
          tunnel: [w4648 w4649] -> w4632
          tunnel: w4628 -> [w4648 _]
          frame False {
            "Humidity temp 2" <- w4648
          }
          frame True {
            n3581 = local read "Humidity temp 2"() -> (w4649:dbl)
          }
        }
        n3582 = local write "RH Numeric:"(w4632) -> ()
      }
    }
    n3583 = local read "Quit"() -> (w4598:bool)
  }
  n3584 = while {
    shift-right: [w4655] -> _
    shift-left: _ -> [w4656]
    shift-right: [w4653] -> _
    shift-left: T20 {"Read Uno"="", "Bytes at Heave Port"=0.0, "UNO COM Port:"="COM9", "UNO COM Port: 2"="COM7", "Residual Due"="", "UNO COM Status 2"=TRUE, "UNO COM Status"=TRUE, "Port 2"=TRUE, "Sway PPR"=6400.0, "Surge PPR"=6400.0, "Heave PPR"=6400.0, "Sway Pitch"=2.0, "Surge Pitch"=3.0, "Heave Pitch"=4.0, "Sway Pulses/mm"=320.0, "Surge Pulses/mm"=1600.0, "Heave Pulses/mm"=1600.0, "inner loop"=0.0, "Read Heave and Surge 2"="", "String 36"="", "Write S"=FALSE, "WriteCC1"=[""], "Heave COM Loop"=0, "LastCom"="", "EXIT"=FALSE, "Error Heave"={"status"=TRUE, "code"=-1073807343, "source"=""}} -> [w4652]
    shift-right: [w4650] -> _
    shift-left: enum16{"init", "MAIN", "Panel Close"}."init" -> [w4651]
    stop <- w4654 stop-if-true
    # "UNO CODE LOGIC"
    n3585 = case shown="\"MAIN\"" w4651 {
      tunnel: w4656 -> [w4670 w4689 w4745 w4747]
      tunnel: [w4665 w4694 w4745 w4747] -> w4655
      tunnel: [_ _ TRUE _] -> w4654
      tunnel: [w4661 w4692 w4743 w4746] -> w4653
      tunnel: w4652 -> [w4667 w4688 w4743 w4746]
      tunnel: [enum16{"init", "MAIN", "Panel Close"}."MAIN" w4683 _ _] -> w4650
      frame "init" {
        n3586 = local read "Com Port 1"() -> (w4657:refnum<visa-resource-name>)
        n3587 = Bundle By Name(cluster=w4667, "UNO COM Port:"=w4657) -> (w4666:T20)
        n3588 = call "Instrument fgv.vi"("Enum"=T31."INIT", "error in (no error) 2"=w4670, "INPUT"=w4666) -> ("error"=w4668:errorcluster, "output"=w4664:T18)  [unwired: 6 in, 1 out]
        n3589 = case shown="Error" w4668 {
          selector: w4668 -> [w4672 _]
          tunnel: [w4672 w4676] -> w4665
          tunnel: w4664 -> [w4671 w4674]
          tunnel: [w4671 w4673] -> w4662
          frame No Error {
          }
          frame Error {
            n3590 = call "Instrument fgv.vi"("Enum"=T31."ERROR INIT", "INPUT"=w4674) -> ("error"=w4677:errorcluster, "output"=w4673:T18)  [unwired: 7 in, 1 out]
            n3591 = call <vilib>:"Clear Errors.vi"("error in (no error)"=w4677) -> ("error out"=w4676:errorcluster)  [unwired: 5 in, 1 out]
          }
        }
        n3592 = local read "LastCom UNO"() -> (w4659:string)
        n3593 = Unbundle By Name(w4662) -> ("Heave COM Status 2"=→"Instrument Status":bool, "Error Heave"=→"Error  2":errorcluster)  [unwired: 1 out]
        n3594 = Bundle By Name(cluster=w4662, "LastCom"=w4659) -> (w4661:T18)
      }
      frame "MAIN" {
        n3595 = Unbundle By Name(w4688) -> ("UNO COM Port: 2"=w4678:refnum<visa-resource-name>)
        n3596 = local read "Com Port 1"() -> (w4679:refnum<visa-resource-name>)
        n3597 = local write "COM Port UNO :"(w4678) -> ()
        n3598 = Equal?(x=w4678, y=w4679) -> (x = y?=w4695:bool)
        n3599 = Bundle By Name(cluster=w4688, "UNO COM Port:"=w4679) -> (w4687:T20)
        n3600 = case shown="True" w4695 {
          tunnel: [w4699 w4716] -> w4694
          tunnel: w4689 -> [w4700 w4722]
          tunnel: w4687 -> [w4698 w4720]
          tunnel: [w4697 w4715] -> w4692
          frame False {
            n3601 = call <vilib>:"Clear Errors.vi"("error in (no error)"=w4700) -> ("error out"=w4696:errorcluster)  [unwired: 5 in, 1 out]
            n3602 = call "Instrument fgv.vi"("Enum"=T31."ERROR INIT", "error in (no error) 2"=w4696, "INPUT"=w4698) -> ("error"=w4702:errorcluster, "output"=w4697:T18)  [unwired: 6 in, 1 out]
            n3603 = call <vilib>:"Clear Errors.vi"("error in (no error)"=w4702) -> ("error out"=w4699:errorcluster)  [unwired: 5 in, 1 out]
          }
          frame True {
            n3604 = call "Instrument fgv.vi"("Enum"=T31."READ", "error in (no error) 2"=w4722, "INPUT"=w4720) -> ("error"=w4721:errorcluster, "output"=w4714:T18)  [unwired: 6 in, 1 out]
            n3605 = Bundle By Name(cluster=w4714, "String 36"="WRITE UNO") -> (w4713:T18)
            n3606 = case shown="True" "Write" {
              selector: "Write" -> [_ w4737]
              tunnel: w4721 -> [w4735 w4742]
              tunnel: [w4735 w4741] -> w4711
              tunnel: w4713 -> [w4734 w4739]
              tunnel: [w4734 w4738] -> w4710
              frame False {
              }
              frame True {
                n3607 = Not(x=w4737) -> (.not. x?=w4736:bool)
                n3608 = local write "Write"(w4736) -> ()
                n3609 = call "Instrument fgv.vi"("Enum"=T31."MANUAL WRITE", "error in (no error) 2"=w4742, "INPUT"=w4739) -> ("error"=w4741:errorcluster, "output"=w4738:T18)  [unwired: 6 in, 1 out]
              }
            }
            n3610 = Array Size(array="Write UNO") -> (size(s)=w4708:i32)
            n3611 = Greater Than 0?(x=w4708) -> (x > 0?=w4707:bool)
            n3612 = call "Instrument fgv.vi"("Enum"=T31."WRITE", "error in (no error) 2"=w4711, "WriteCC1"="Write UNO", "INPUT"=w4710) -> ("error"=w4718:errorcluster, "WriteCC1 2"=w4709:string[], "output"=w4717:T18)  [unwired: 5 in]
            n3613 = case shown="True" w4707 {
              tunnel: w4709 -> [_ w4724]
              frame False {
              }
              frame True {
                n3614 = local write "Write UNO"(w4724) -> ()
              }
            }
            n3615 = case shown="Error" w4718 {
              selector: w4718 -> [w4725 w4728]
              tunnel: w4717 -> [w4726 w4733]
              tunnel: [w4726 w4732] -> w4715
              tunnel: [w4725 w4730] -> w4716
              frame No Error {
              }
              frame Error {
                n3616 = call <vilib>:"Clear Errors.vi"("error in (no error)"=w4728) -> ("error out"=w4727:errorcluster)  [unwired: 5 in, 1 out]
                n3617 = call "Instrument fgv.vi"("Enum"=T31."ERROR INIT", "error in (no error) 2"=w4727, "INPUT"=w4733) -> ("error"=w4731:errorcluster, "output"=w4732:T18)  [unwired: 6 in, 1 out]
                n3618 = call <vilib>:"Clear Errors.vi"("error in (no error)"=w4731) -> ("error out"=w4730:errorcluster)  [unwired: 5 in, 1 out]
              }
            }
            n3619 = Unbundle By Name(w4715) -> ("LastCom"=→"LastCom UNO":string, "Read Heave and Surge"=→"Read UNO":string)
          }
        }
        n3620 = Unbundle By Name(w4692) -> ("Heave COM Status 2"=w4693:bool, "Heave COM Status"=w4682:bool, "Error Heave"=w4680:errorcluster, "Bytes at Heave Port"=→"Bytes at Humidity Port":dbl)
        n3621 = Not(x=w4682) -> (.not. x?=w4690:bool)
        n3622 = Not(x=w4693) -> (.not. x?=w4681:bool)
        n3623 = local write "Instrument Status"(w4690) -> ()
        n3624 = local write "Error  2"(w4680) -> ()
        n3625 = local write "Port 1a"(w4682) -> ()
        n3626 = local read "Quit"() -> (w4684:bool)
        n3627 = local write "COM Status"(w4681) -> ()
        n3628 = Select(t=enum16{"init", "MAIN", "Panel Close"}."Panel Close", s=w4684, f=enum16{"init", "MAIN", "Panel Close"}."MAIN") -> (s? t:f=w4683:enum16{"init", "MAIN", "Panel Close"})
      }
      frame "Panel Close" {
      }
      frame Default {
      }
    }
  }
